vi "UHR-Fleezers Control (host) - 10.3.vi"() -> ()   [LabVIEW 2010] (continued)
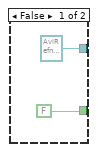
[diagram p2: hidden frame]
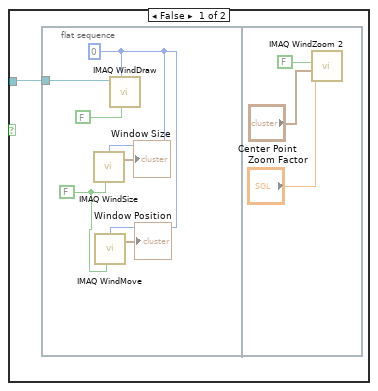
[diagram p5: hidden frame]
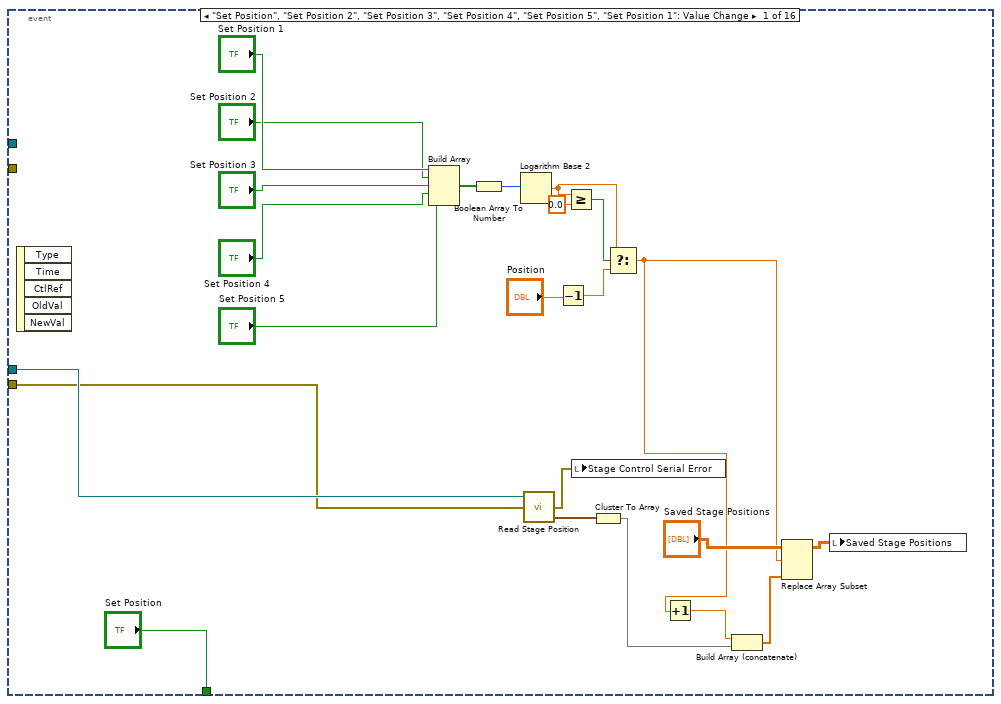
[diagram p11: hidden frame]
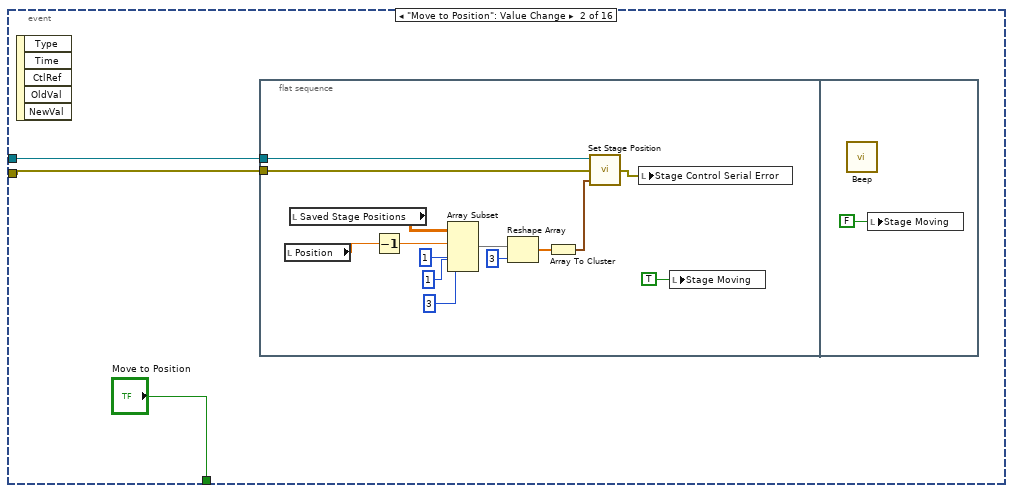
[diagram p12: hidden frame]
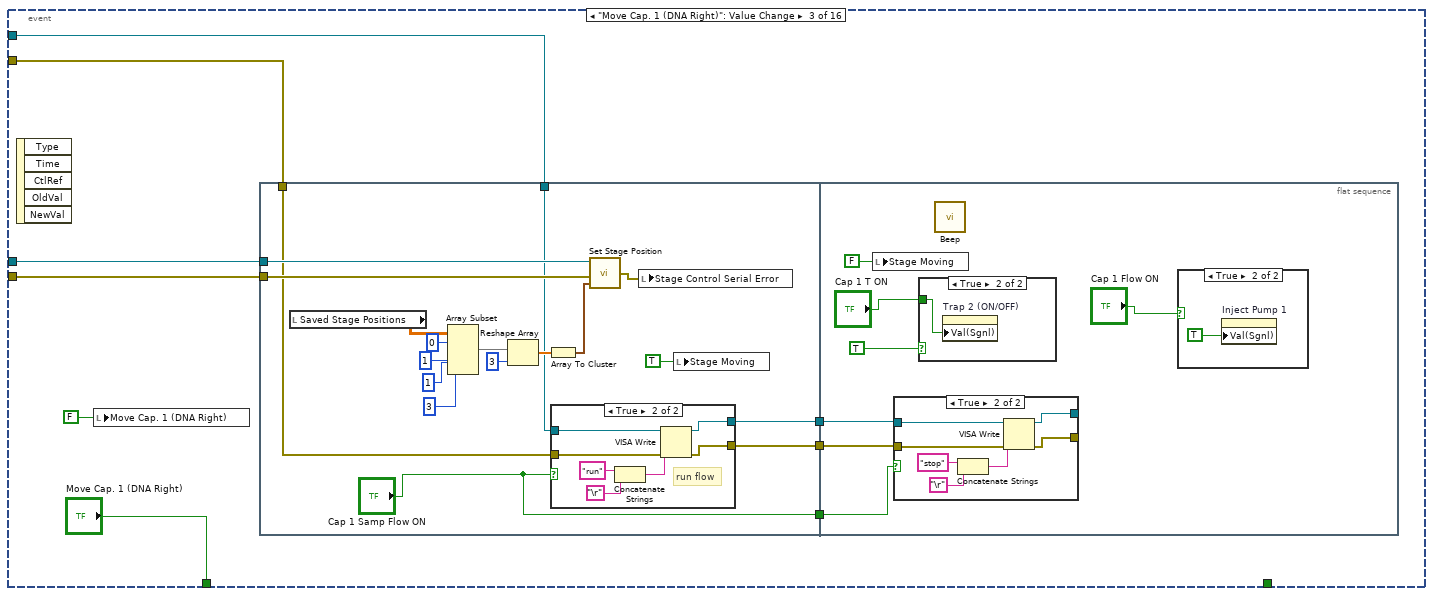
[diagram p13: hidden frame]
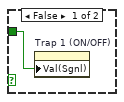
[diagram p17: hidden frame]
                          n1976 = local write "BD 2 Frequency 1 (MHz)"(w8359) -> ()
                          n1977 = local write "BD 1 Frequency 1 (MHz)"(w8361) -> ()
                        }
                      }
                    }
                    frame True {
                    }
                  }
                }
                event Mouse Up {
                  n1978 = event-data() -> ("Button"=w8364:u16)  [unwired: 8 out]
                  n1979 = case shown="3" w8364 {
                    tunnel: [FALSE TRUE] -> w8365
                    frame 0, Default {
                    }
                    frame 3 {
                      n1980 = local write "Manipulating Trap"(FALSE ("Manipulating Trap")) -> ()
                    }
                  }
                }
              }
            }
          }
        }
      }
      event Mouse Move {
        n1981 = event-data() -> ()  [unwired: 6 out]
      }
    }
    n1982 = local read "Stop All"() -> (w8186:bool)
    n1983 = node-c288() -> ()  [unwired: 2 out]
  }
  n1984 = disable-structure shown="Disabled" {
    frame Disabled {
      n1985 = flat-sequence "Video" {
        tunnel: [w8378] -> w8369
        tunnel: w8369 -> [w8419]
        frame #0 {
          n1986 = while {
            stop <- w8371 continue-if-true
            n1987 = call "Close Video Capture.vi"() -> ("error code OUT"=w8373:i32)
            n1988 = Equal?(x=w8373, y=0) -> (x = y?=w8371:bool)
          }
          n1989 = local write "Stop All"(FALSE ("Stop All")) -> ()
        }
        frame #1 {
          n1990 = call "DMR_Init.vi"() -> ()  [unwired: 3 out]
        }
        frame #2 {
          # "Setting the destination format to Mono8 makes sure that the image can be displayed in the intensity plot."
          n1991 = call "DMR_GetDevice.vi"("search string IN"="DE019116701") -> ("device handle OUT"=w8396:i32)  [unwired: 4 in, 2 out]
          n1992 = call "DMR_OpenDevice.vi"("device handle IN"=w8396) -> ("driver handle OUT"=w8379:i32)  [unwired: 4 out]
          n1993 = call "DMR_FindList.vi"("flags IN"=u32 0 ("flags"), "list name IN"="" ("String"), "list type IN"=T47."camera descriptions", "driver handle IN"=w8379) -> ("list handle OUT"=w8382:i32)  [unwired: 2 out]
          n1994 = call "DMR_FindList.vi"("flags IN"=u32 0 ("flags"), "list name IN"="Base", "list type IN"=T47."setting", "driver handle IN"=w8379) -> ("list handle OUT"=w8380:i32)  [unwired: 2 out]
          n1995 = call "OBJ_GetHandle.vi"("object name IN"="VideoStandard", "list handle IN"=w8382) -> ("object handle OUT"=w8376:i32)  [unwired: 3 out]
          n1996 = call "OBJ_GetHandle.vi"("object name IN"="PixelFormat", "list handle IN"=w8380) -> ("object handle OUT"=w8390:i32)  [unwired: 3 out]
          n1997 = call "OBJ_SetS.vi"("value index IN"=0, "value IN"="NTSC M", "object handle IN"=w8376) -> ()  [unwired: 2 out]
          n1998 = call "OBJ_SetS.vi"("value index IN"=0, "value IN"="Mono8" ("value"), "object handle IN"=w8390) -> ()  [unwired: 2 out]
          n1999 = call "OBJ_GetHandle.vi"("object name IN"="VideoChannel", "list handle IN"=w8380) -> ("object handle OUT"=w8386:i32)  [unwired: 3 out]
          n2000 = while {
            tunnel: [w8401] -> w8378
            tunnel: w8379 -> [w8398]
            stop <- w8399 continue-if-true
            n2001 = call "DMR_ImageRequestSingle.vi"("request control IN"=0, "driver handle IN"=w8398) -> ("error code OUT"=w8400:i32, "driver handle OUT"=w8401:i32)  [unwired: 2 out]
            n2002 = Equal To 0?(x=w8400) -> (x = 0?=w8399:bool)
          }
          n2003 = call "OBJ_SetI.vi"("value index IN"=0, "value IN"=3 ("Video channel"), "object handle IN"=w8386) -> ()  [unwired: 2 out]
        }
        frame #3 {
          w8407 = T17 0 items=["Grayscale (U8)", "Grayscale (I16)", "Grayscale (SGL)", "Complex (CSG)", "RGB (U32)", "HSL (U32)", "RGB (U64)"] ("Image Type")
          w8415 = T17 0 items=["Grayscale (U8)", "Grayscale (I16)", "Grayscale (SGL)", "Complex (CSG)", "RGB (U32)", "HSL (U32)", "RGB (U64)"] ("Image Type")
          n2004 = for "Create Greyscale map" {
            N: 256 -> [_]
            tunnel: [w8421] -> w8404 mode=indexing
            workers-P: _ -> [_]
            i -> [w8424]
            n2005 = To Unsigned Byte Integer(number=w8424) -> (unsigned 8bit integer=w8420:u8)
            n2006 = Join Numbers(hi=w8420, lo=w8420) -> ((hi.lo)=w8423:u16)
            n2007 = Join Numbers(hi=w8420, lo=w8420) -> ((hi.lo)=w8422:u16)
            n2008 = Join Numbers(hi=w8423, lo=w8422) -> ((hi.lo)=w8421:u32)
          }
          n2009 = call "IMAQ Create"("Image Name"="Scaled video", "Image Type"=w8407) -> ("New Image"=w8406:T2)  [unwired: 2 in, 2 out]
          n2010 = call "IMAQ Create"("Image Name"="Main video", "Image Type"=w8415) -> ("New Image"=w8416:T2)  [unwired: 2 in, 2 out]
          n2011 = node-c288(0 ("Processor")) -> (w8414:T23)  [unwired: 3 out]
          n2012 = Initialize Array(u32 0 ("Window Number (0...15)"), 480 ("dimension size"), 640 ("dimension size")) -> (w8409:u32[][])
          n2013 = timed-loop {
            tunnel: w8419 -> [w8441]
            tunnel: [w8440] -> w8418
            tunnel: w8416 -> [w8439]
            timing: w8414 -> [_]
            timing-out: [_] -> w8413
            tunnel: w8409 -> [w8428]
            tunnel: w8406 -> [w8426]
            tunnel: w8404 -> [w8425]
            stop <- w8427 stop-if-true
            # "This block performs the \nactual image capture."
            n2014 = node-c288() -> ()  [unwired: 2 out]
            n2015 = local read "Stop All"() -> (w8427:bool)
            n2016 = Reciprocal(x="Video Capture Rate (Hz)") -> (1/x=w8431:dbl)
            n2017 = Multiply(x=w8431, y=1000.0) -> (x*y=w8429:dbl)
            n2018 = call "DMR_ImageRequestWaitFor.vi"("queue number IN"=0, "timeout(ms) IN"=500, "driver handle IN"=w8441) -> ("error code OUT"=w8445:i32, "request number OUT"=w8442:i32, "driver handle OUT"=w8443:i32)
            n2019 = feedback #31(T48 refnum ("Avi Refnum")) -> (w8433:T48)
            n2020 = case shown="True" "New Video File" {
              tunnel: [T48 refnum ("Avi Refnum") w8462] -> w8435
              tunnel: [FALSE TRUE] -> w8436
              tunnel: w8433 -> [_ w8458]
              frame False {
              }
              frame True {
                n2021 = call "Create new save file.vi"("Ext"=".avi" ("string"), "Index In"="Video Index") -> ("Path Out"=w8454:path, "Index Out"=w8455:dbl)  [unwired: 1 in]
                "Path Out" <- w8454
                n2022 = Not Equal?(x=w8458, y=T48 refnum ("Avi Refnum")) -> (x != y?=w8459:bool)
                n2023 = Increment(x=w8455) -> (x+1=w8464:dbl)
                n2024 = case shown="True" w8459 {
                  tunnel: w8458 -> [_ w8465]
                  frame False {
                  }
                  frame True {
                    n2025 = call "IMAQ AVI Close"("Avi Refnum"=w8465) -> ()  [unwired: 1 in, 10 out]
                  }
                }
                n2026 = local write "Video Index"(w8464) -> ()
                n2027 = call "IMAQ AVI Create"("Frames Per Second"=u32 30, "AVI Path"=w8454) -> ("Avi Refnum"=w8462:T48)  [unwired: 5 in, 4 out]
              }
            }
            n2028 = Equal To 0?(x=w8445) -> (x = 0?=w8444:bool)
            n2029 = Select(t=w8435, s=w8436, f=w8433) -> (s? t:f=w8434:T48)
            n2030 = feedback-in #31(w8434) -> ()
            n2031 = case shown="True" w8444 {
              tunnel: w8443 -> [w8466 w8491]
              tunnel: w8442 -> [_ w8490]
              tunnel: [w8466 w8487] -> w8440
              tunnel: w8439 -> [_ w8471]
              tunnel: w8428 -> [_ w8475]
              tunnel: w8434 -> [_ w8473]
              tunnel: w8426 -> [_ w8468]
              tunnel: w8425 -> [_ w8467]
              frame False {
              }
              frame True {
                w8481 = u32 0 ("X-offset IN")
                n2032 = call "DMR_GetImageRequestBufferData.vi"("driver handle IN"=w8491, "request number IN"=w8490) -> ("width OUT"=w8480:i32, "height OUT"=w8479:i32, "driver handle OUT"=w8486:i32, "request number OUT"=w8485:i32, "bytes per pixel OUT"=w8482:i32)  [unwired: 13 out]
                n2033 = call "DMR_GetImageRequestBufferImageData.vi"("driver handle IN"=w8486, "request number IN"=w8485, "bytes per pixel IN"=w8482, "X-offset IN"=w8481, "Y-offset IN"=w8481, "height IN"=w8479, "width IN"=w8480) -> ("driver handle OUT"=w8484:u32, "request number OUT"=w8483:u32, "image OUT"=w8476:u32[][])  [unwired: 10 out]
                n2034 = call "DMR_ImageRequestUnlock.vi"("request number IN"=w8483, "driver handle IN"=w8484) -> ("driver handle OUT"=w8489:i32)  [unwired: 1 in, 2 out]
                n2035 = case shown="True" "Averaging" {
                  tunnel: w8476 -> [w8527 w8532]
                  tunnel: [w8527 w8531] -> w8472
                  tunnel: w8475 -> [_ w8529]
                  frame False {
                  }
                  frame True {
                    (unwired) 1
                    w8537 = 1
                    n2036 = feedback #32(w8529) -> (w8528:u32[][])
                    n2037 = Add(x=w8532, y=w8528) -> (x+y=w8533:u32[][])
                    n2038 = Select(t=w8529, s="Reset Averaging", f=w8533) -> (s? t:f=w8535:u32[][])
                    n2039 = feedback-in #32(w8535) -> ()
                    n2040 = feedback #33(w8537) -> (w8530:i32)
                    n2041 = Divide(x=w8533, y=w8530) -> (x/y=w8534:dbl[][])
                    n2042 = Increment(x=w8530) -> (x+1=w8538:i32)
                    n2043 = To Unsigned Long Integer(number=w8534) -> (unsigned 32bit integer=w8531:u32[][])
                    n2044 = Select(t=w8537, s="Reset Averaging", f=w8538) -> (s? t:f=w8536:i32)
                    n2045 = feedback-in #33(w8536) -> ()
                  }
                }
                n2046 = call "DMR_ImageRequestSingle.vi"("request control IN"=0, "driver handle IN"=w8489) -> ("driver handle OUT"=w8487:i32)  [unwired: 3 out]
                n2047 = disable-structure shown="Disabled" {
                  disable-tunnel: w8472 -> [w8504 _]
                  disable-tunnel: w8468 -> [w8503 _]
                  frame Disabled {
                    n2048 = To Double Precision Float(number=w8504) -> (double precision float=w8502:dbl[][])
                    n2049 = In Range and Coerce(upper limit="Intensity Upper", x=w8502, lower limit="Intensity Lower") -> (coerced(x)=w8501:dbl[][])  [unwired: 1 out]
                    n2050 = Subtract(x="Intensity Upper", y="Intensity Lower") -> (x-y=w8498:dbl)
                    n2051 = Subtract(x=w8501, y="Intensity Lower") -> (x-y=w8499:dbl[][])
                    n2052 = Divide(x=w8499, y=w8498) -> (x/y=w8500:dbl[][])
                    n2053 = Multiply(x=255.0, y=w8500) -> (x*y=w8496:dbl[][])
                    n2054 = To Unsigned Byte Integer(number=w8496) -> (unsigned 8bit integer=w8505:u8[][])
                    n2055 = call "IMAQ ArrayToImage"("Image Pixels (U8)"=w8505, "Image"=w8503) -> ("Image Out"=w8492:T2)  [unwired: 4 in, 5 out]
                    n2056 = First Call?() -> (First Call?: T/F=w8493:bool)
                    n2057 = case shown="True" w8493 {
                      tunnel: w8492 -> [w8506 w8517]
                      frame False {
                        n2058 = flat-sequence {
                          tunnel: w8506 -> [w8512]
                          frame #0 {
                            w8509 = FALSE ("Get/Set Status? (Set)")
                            w8508 = 0 ("Window Number (0...15)")
                            n2059 = call "IMAQ WindSize"("Get/Set Status? (Set)"=w8509, "Window Number"=w8508) -> ("Width & Height out"=→"Window Size":cluster{"Width":i32, "Height":i32})  [unwired: 4 in, 2 out]
                            n2060 = call "IMAQ WindMove"("Window Number (0...15)"=w8508, "Get/Set Status? (Set)"=w8509) -> ("Coordinates (screen)"=→"Window Position":cluster{"X Position":i32, "Y Position":i32})  [unwired: 3 in, 1 out]
                            n2061 = call "IMAQ WindDraw"("Resize to Image Size? (Y)"=FALSE, "Window Number (0...15)"=w8508, "Image"=w8512) -> ()  [unwired: 7 in, 2 out]
                          }
                          frame #1 {
                            n2062 = call "IMAQ WindZoom 2"("Center Point"="Center Point", "Zoom to Fit? (False)"=FALSE, "Zoom Factor"="Zoom Factor") -> ()  [unwired: 5 in, 4 out]
                          }
                        }
                      }
                      frame True {
                        n2063 = flat-sequence {
                          tunnel: w8517 -> [w8520]
                          tunnel: [w8518] -> w8516
                          tunnel: w8516 -> [w8522]
                          frame #0 {
                            w8519 = TRUE ("Resize to Image Size? (Y)")
                            w8518 = 0 ("Window Number (0...15)")
                            n2064 = call "IMAQ WindNonTearing"("Window Number"=w8518, "NonTearing? (True)"=w8519) -> ()  [unwired: 8 in, 2 out]
                            n2065 = call "IMAQ WindDraw"("Resize to Image Size? (Y)"=w8519, "Window Number (0...15)"=w8518, "Image"=w8520) -> ()  [unwired: 7 in, 2 out]
                          }
                          frame #1 {
                            n2066 = call "IMAQ WindSize"("Scrollbars? (N)"=FALSE, "Width & Height"="Initial Window Size", "Window Number"=w8522) -> ()  [unwired: 3 in, 3 out]
                            n2067 = call "IMAQ WindMove"("Window Number (0...15)"=w8522, "Coordinates (screen)"="Initial Window Position") -> ()  [unwired: 3 in, 2 out]
                          }
                        }
                      }
                    }
                  }
                  frame Enabled {
                  }
                }
                n2068 = To Unsigned Byte Integer(number=w8472) -> (unsigned 8bit integer=w8470:u8[][])
                n2069 = call "IMAQ ArrayToImage"("Image Pixels (U8)"=w8470, "Image"=w8471) -> ("Image Out"=w8469:T2)  [unwired: 4 in, 5 out]
                "Primary Video Display" <- w8469
                n2070 = case shown="True" "Save Video" {
                  tunnel: w8473 -> [_ w8526]
                  tunnel: w8469 -> [_ w8525]
                  frame False {
                  }
                  frame True {
                    n2071 = call "IMAQ AVI Write Frame"("Image"=w8525, "Avi Refnum"=w8526) -> ()  [unwired: 2 in, 8 out]
                  }
                }
                n2072 = case shown="True" "Save Image" {
                  tunnel: w8470 -> [_ w8541]
                  tunnel: w8467 -> [_ w8540]
                  frame False {
                  }
                  frame True {
                    n2073 = call <vilib>:"Flatten Pixmap.vi"("colors"=w8540, "8-bit pixmap"=w8541) -> ("image data"=w8547:T49)  [unwired: 4 in, 5 out]
                    n2074 = call "Create new save file.vi"("Insert"="video_frame_" ("string"), "Ext"=".bmp" ("string"), "Index In"="Image Index") -> ("Path Out"=w8543:path, "Index Out"=w8548:dbl)
                    n2075 = Increment(x=w8548) -> (x+1=w8542:dbl)
                    n2076 = local write "Image Index"(w8542) -> ()
                    n2077 = call <vilib>:"Write BMP File.vi"("image data"=w8547, "path to BMP file"=w8543) -> ()  [unwired: 1 in, 9 out]
                  }
                }
              }
            }
            n2078 = node-c288(w8429) -> ()  [unwired: 1 out]
          }
          n2079 = node-c288(w8413) -> ()  [unwired: 1 out]
          n2080 = call "DMR_CloseDevice.vi"("driver handle IN"=w8418) -> ()  [unwired: 1 in, 4 out]
        }
        frame #4 {
          n2081 = call "DMR_Close.vi"() -> ()  [unwired: 1 out]
        }
      }
    }
    frame Enabled {
    }
  }
  n2082 = timed-loop "Oscillate AOD (debugging)" {
    tunnel: w8 -> [w8554]
    tunnel: [w8553] -> w52
    timing: w47 -> [_]
    timing-out: [_] -> w46
    stop <- w8553 stop-if-true
    n2083 = node-c288() -> ()  [unwired: 2 out]
    n2084 = event shown="[0] \"Oscillate Set 1\", \"Fish for Tether\": Value Change" {
      selector: _ -> [_ _ _]
      dyn-events: _ -> [_ _ _]
      timeout: _ -> [_ _ _]
      tunnel: w8554 -> [w8561 _ _]
      tunnel: [FALSE ("Stop All") _ w8830] -> w8553
      event "Oscillate Set 1", "Fish for Tether": Value Change {
        n2085 = event-data() -> ()  [unwired: 6 out]
        n2086 = local read "Oscillate Set 1"() -> (w8560:bool)
        n2087 = Or(x=w8560, y="Fish for Tether") -> (x .or. y?=w8558:bool)
        n2088 = case shown="True" w8558 {
          tunnel: w8561 -> [_ w8564]
          tunnel: "Fish for Tether" -> [_ w8563]
          frame False {
          }
          frame True {
            n2089 = case shown="False" w8563 {
              frame False {
              }
              frame True {
                n2090 = local write "Scan axis 2"(TRUE) -> ()
                n2091 = local write "Tether"(FALSE ("Tether")) -> ()
              }
            }
            n2092 = node-c288(i64 50 ("Period")) -> (w8566:T23)  [unwired: 3 out]
            n2093 = timed-loop "Oscillate AOD" {
              timing: w8566 -> [_]
              timing-out: [_] -> w8565
              tunnel: w8564 -> [w8576]
              tunnel: w8563 -> [w8575]
              i -> [w8578]
              stop <- w8574 stop-if-true
              n2094 = node-c288() -> (w8577:i64)  [unwired: 1 out]
              n2095 = flat-sequence {
                tunnel: w8578 -> [w8605]
                tunnel: w8577 -> [w8604]
                tunnel: w8576 -> [w8585]
                tunnel: w8575 -> [w8588]
                tunnel: [w8588] -> w8573
                tunnel: [w8587] -> w8572
                tunnel: [w8584] -> w8571
                tunnel: [w8581] -> w8569
                tunnel: w8573 -> [w8641]
                tunnel: w8572 -> [w8639]
                tunnel: w8571 -> [w8638]
                tunnel: [w8637] -> w8570
                tunnel: w8569 -> [w8636]
                tunnel: [w8705] -> w8574
                tunnel: w8570 -> [w8703]
                frame #0 {
                  n2096 = Divide(x=w8604, y=i64 1000) -> (x/y=w8599:dbl)
                  n2097 = Multiply(x=w8599, y=w8605) -> (x*y=w8601:dbl)
                  n2098 = Multiply(x="Osc. freq. (Hz)", y=6.283185307179586) -> (x*y=w8602:dbl)
                  n2099 = Multiply(x=w8602, y=w8601) -> (x*y=w8583:dbl)
                  n2100 = local read "BD 1 Frequency 2 (MHz)"() -> (w8586:dbl)
                  n2101 = local read "BD 1 Frequency 1 (MHz)"() -> (w8579:dbl)
                  n2102 = case shown="False" w8588 {
                    tunnel: w8583 -> [w8611 w8617]
                    tunnel: w8586 -> [_ w8628]
                    tunnel: [w8608 w8623] -> w8589
                    tunnel: [FALSE w8620] -> w8584
                    tunnel: [0.0 w8613] -> w8581
                    tunnel: w8579 -> [_ w8612]
                    frame False {
                      n2103 = Sine(x=w8611) -> (sin(x)=w8609:dbl)
                      n2104 = Multiply(x=w8609, y="Osc. amp. (MHz)") -> (x*y=w8608:dbl)
                    }
                    frame True {
                      n2105 = Cosine(x=w8617) -> (cos(x)=w8631:dbl)
                      n2106 = Subtract(x=w8628, y=w8612) -> (x-y=w8627:dbl)
                      n2107 = Decrement(x=w8631) -> (x-1=w8630:dbl)
                      n2108 = Subtract(x=w8627, y="Closest Delta (MHz)") -> (x-y=w8624:dbl)
                      n2109 = Divide(x=w8630, y=-2.0) -> (x/y=w8625:dbl)
                      n2110 = Multiply(x=w8625, y=w8624) -> (x*y=w8623:dbl)
                      n2111 = local read "Vec Mean of T1 T2"() -> (w8619:dbl[])
                      n2112 = Greater?(x=w8619, y="Stop F (pN)") -> (0:w8621:bool[])
                      n2113 = Or Array Elements(Boolean array=w8621) -> (logical OR=w8620:bool)
                      n2114 = Divide(x=w8617, y=6.283185307179586) -> (x/y=w8616:dbl)
                      n2115 = Round Toward +Infinity(x=w8616) -> (ceil(x): smallest int >= x=w8613:dbl)
                      "Attempts" <- w8613
                      n2116 = Greater?(x=w8613, y="Attempt Limit") -> (0:w8615:bool)
                      n2117 = case shown="True" w8615 {
                        frame False {
                        }
                        frame True {
                          n2118 = local write "Fish for Tether"(FALSE ("Fish for Tether")) -> ()
                          n2119 = call <vilib>:"Beep.vi"() -> ()  [unwired: 3 in, 9 out]
                          n2120 = local read "Messages"() -> (w8633:string)
                          n2121 = call "Update messages.vi"("Message to add"="Tether fishing timeout." ("Messages"), "Old message string"=w8633) -> ("New message string"=→"Messages":string)
                        }
                      }
                    }
                  }
                  n2122 = local read "BD 2 Frequency 1 (MHz)"() -> (w8590:dbl)
                  n2123 = Select(t=w8579, s="Scan axis 2", f=w8590) -> (s? t:f=w8593:dbl)
                  n2124 = Add(x=w8589, y=w8593) -> (x+y=w8587:dbl)
                  n2125 = Select(t=w8587, s="Scan axis 2", f=w8579) -> (s? t:f=w8580:dbl)
                  n2126 = Select(t=w8590, s="Scan axis 2", f=w8587) -> (s? t:f=w8595:dbl)
                  n2127 = local read "Y RF Frequency Limits (MHz)"() -> (w8591:T16)
                  n2128 = local read "X RF Frequency Limits (MHz)"() -> (w8592:T16)
                  n2129 = local read "BD 1 Frequency 3 (MHz)"() -> (w8598:dbl)
                  n2130 = local read "BD 2 Frequency 2 (MHz)"() -> (w8597:dbl)
                  n2131 = local read "BD 2 Frequency 3 (MHz)"() -> (w8596:dbl)
                  n2132 = call "set RF board frequency - interlace.vi"("Board 2 Frequency Limits"=w8591, "Board 1 Frequency Limits"=w8592, "FPGA VI Reference In"=w8585, "Board 2 Frequency 3 (MHz)"=w8596, "Board 1 Frequency 3 (MHz)"=w8598, "Board 2 Frequency 2 (MHz)"=w8597, "Board 2 Frequency 1 (MHz)"=w8595, "Board 1 Frequency 2 (MHz)"=w8586, "Board 1 Frequency 1  (MHz)"=w8580) -> ()  [unwired: 1 in, 2 out]
                }
                frame #1 {
                  n2133 = And(x=w8641, y=w8638) -> (x .and. y?=w8640:bool)
                  n2134 = case "Only if were fishing and now formed tether" shown="False" w8640 {
                    tunnel: w8639 -> [w8643 w8655]
                    tunnel: [w8642 w8654] -> w8637
                    tunnel: w8636 -> [_ w8650]
                    frame False {
                      n2135 = local read "Fish for Tether"() -> (w8642:bool)
                      n2136 = case shown="False" w8642 {
                        tunnel: w8643 -> [_ _]
                        frame False {
                        }
                        frame True {
                        }
                      }
                    }
                    frame True {
                      w8654 = FALSE ("Fish for Tether")
                      n2137 = call <vilib>:"Beep.vi"() -> ()  [unwired: 3 in, 9 out]
                      n2138 = Number To Decimal String(number=w8650, width (-)=i16 1) -> (decimal integer string=w8648:string)
                      n2139 = case shown="\"1\", Default" "Then..." {
                        selector: "Then..." -> [_ w8658]
                        tunnel: w8655 -> [w8657 _]
                        frame "1", Default {
                          n2140 = property on="BD 1 Frequency 1 (MHz)" class="DigNum (strict)"("Val(Sgnl)"=w8657) -> ()  [unwired: 2 in, 2 out]
                        }
                        frame "2", "3", "4", "5", "6" {
                          n2141 = flat-sequence {
                            tunnel: w8658 -> [w8660]
                            frame #0 {
                              n2142 = property on="Trap Delta (MHz)" class="DigNum (strict)"("Val(Sgnl)"="Move to Delta 1 (MHz)") -> ()  [unwired: 2 in, 2 out]
                            }
                            frame #1 {
                              n2143 = case shown="\"5\", \"6\"" w8660 {
                                selector: w8660 -> [w8663 w8673 _]
                                frame "3", "4" {
                                n2144 = flat-sequence {
                                tunnel: w8663 -> [w8664]
                                tunnel: [w8664] -> w8661
                                tunnel: [w8666] -> w8662
                                tunnel: w8661 -> [w8666]
                                tunnel: w8662 -> [w8670]
                                frame #0 {
                                n2145 = property on="Green Laser ON/Interlacing" class="Bool (strict)"("Val(Sgnl)"=TRUE ("Value (Signaling)")) -> ()  [unwired: 2 in, 2 out]
                                }
                                frame #1 {
                                n2146 = Multiply(x="Wait Before Save (s)", y=u32 1000 ("x")) -> (x*y=w8668:u32)
                                n2147 = Wait (ms)(milliseconds to wait=w8668) -> ()  [unwired: 1 out]
                                }
                                frame #2 {
                                n2148 = property on="Start Saving" class="Bool (strict)"("Value"=TRUE ("Start Saving")) -> ()  [unwired: 2 in, 2 out]
                                n2149 = case shown="\"4\"" w8670 {
                                frame Default {
                                }
                                frame "4" {
                                n2150 = property on="Fl. Triggered..." class="Bool (strict)"("Val(Sgnl)"=TRUE ("Value (Signaling)")) -> ()  [unwired: 2 in, 2 out]
                                }
                                }
                                }
                                }
                                }
                                frame "5", "6" {
                                n2151 = stacked-sequence {
                                tunnel: w8673 -> [_ _ _ _ _ _ _ _ w8690 _ _]
                                frame #0 {
                                n2152 = Replace Array Subset(array=u32[] [0] ("Index Values"), new element="Raster Set Upon Tether", index=0) -> (w8674:u32[])
                                n2153 = property on="Saved AOD Raster Scan Parameter Sets" class="Arr (strict)"("Index Values"=w8674) -> ()  [unwired: 2 in, 2 out]
                                }
                                frame #1 {
                                n2154 = Wait (ms)(milliseconds to wait=u32 500) -> ()  [unwired: 1 out]
                                }
                                frame #2 {
                                n2155 = property on="Load parameters" class="Bool (strict)"("Val(Sgnl)"=TRUE ("Value (Signaling)")) -> ()  [unwired: 2 in, 2 out]
                                }
                                frame #3 {
                                n2156 = Wait (ms)(milliseconds to wait=u32 500) -> ()  [unwired: 1 out]
                                }
                                frame #4 {
                                n2157 = property on="Trap Raster Scan" class="Bool (strict)"("Val(Sgnl)"=TRUE ("Value (Signaling)")) -> ()  [unwired: 2 in, 2 out]
                                }
                                frame #5 {
                                n2158 = Wait (ms)(milliseconds to wait=u32 2000) -> ()  [unwired: 1 out]
                                }
                                frame #6 {
                                n2159 = while {
                                stop <- w8685 stop-if-true
                                n2160 = local read "Raster Scanning..."() -> (w8684:bool)
                                n2161 = local read "Saving..."() -> (w8687:bool)
                                n2162 = Wait (ms)(milliseconds to wait=u32 100) -> ()  [unwired: 1 out]
                                n2163 = Not(x=w8687) -> (.not. x?=w8686:bool)
                                n2164 = Not(x=w8684) -> (.not. x?=w8683:bool)
                                n2165 = And(x=w8686, y=w8683) -> (x .and. y?=w8685:bool)
                                }
                                }
                                frame #7 {
                                n2166 = property on="Trap Delta (MHz)" class="DigNum (strict)"("Val(Sgnl)"="Move to Delta 2 (MHz)") -> ()  [unwired: 2 in, 2 out]
                                }
                                frame #8 {
                                n2167 = local read "Tether"() -> (w8691:bool)
                                n2168 = case shown="True" w8691 {
                                tunnel: w8690 -> [_ w8692]
                                frame False {
                                }
                                frame True {
                                n2169 = flat-sequence {
                                tunnel: w8692 -> [w8694]
                                frame #0 {
                                n2170 = Wait (ms)(milliseconds to wait=u32 500) -> ()  [unwired: 1 out]
                                }
                                frame #1 {
                                n2171 = case shown="\"6\"" w8694 {
                                frame Default {
                                }
                                frame "6" {
                                n2172 = property on="Green Laser ON/Interlacing" class="Bool (strict)"("Val(Sgnl)"=TRUE ("Green Laser ON/Interlacing")) -> ()  [unwired: 2 in, 2 out]
                                }
                                }
                                }
                                frame #2 {
                                n2173 = Wait (ms)(milliseconds to wait=u32 500) -> ()  [unwired: 1 out]
                                }
                                frame #3 {
                                n2174 = local write "Start Saving"("Save at end (5, 6)") -> ()
                                }
                                }
                                }
                                }
                                }
                                frame #9 {
                                n2175 = local read "Bead Sep. Int. Time (s)"() -> (w8700:dbl)
                                n2176 = Multiply(x=w8700, y=1000.0) -> (x*y=w8699:dbl)
                                n2177 = Wait (ms)(milliseconds to wait=w8699) -> ()  [unwired: 1 out]
                                }
                                frame #10 {
                                n2178 = property on="Rescale on Mean" class="Bool (strict)"("Val(Sgnl)"=TRUE ("Value (Signaling)")) -> ()  [unwired: 2 in, 2 out]
                                }
                                }
                                }
                                frame "2", Default {
                                }
                              }
                            }
                          }
                        }
                      }
                      n2179 = Concatenate Strings("Formed tether in ", w8648, " attempt(s)." ("string")) -> (w8645:string)
                      n2180 = local read "Messages"() -> (w8652:string)
                      n2181 = local write "Fish for Tether"(w8654) -> ()
                      n2182 = call "Update messages.vi"("Message to add"=w8645, "Old message string"=w8652) -> ("New message string"=w8651:string)
                      n2183 = local write "Messages"(w8651) -> ()
                      n2184 = Get Date/Time In Seconds() -> (seconds since 1Jan1904=→"Time tether formed":timestamp)
                      "Tether" <- "Tether Alarm?"
                    }
                  }
                }
                frame #2 {
                  n2185 = local read "Oscillate Set 1"() -> (w8704:bool)
                  n2186 = local read "Stop All"() -> (w8706:bool)
                  n2187 = Not Or(1:w8703, 2:w8704) -> (0:w8702:bool)
                  n2188 = Compound Arithmetic op=OR(w8706, w8702) -> (w8705:bool)
                }
              }
              n2189 = node-c288() -> ()  [unwired: 2 out]
            }
            n2190 = node-c288(w8565) -> ()  [unwired: 1 out]
          }
        }
      }
      event "Fl. Triggered...": Value Change {
        n2191 = event-data() -> ()  [unwired: 7 out]
        n2192 = case shown="True" "Fl. Triggered..." {
          frame False {
          }
          frame True {
            n2193 = node-c288() -> (w8718:T23)  [unwired: 4 out]
            n2194 = timed-loop {
              timing: w8718 -> [_]
              timing-out: [_] -> w8717
              tunnel: "Action" -> [w8722]
              shift-right: [w8719] -> _
              shift-left: u8 255 -> [w8721]
              stop <- w8723 stop-if-true
              n2195 = node-c288() -> ()  [unwired: 2 out]
              n2196 = flat-sequence {
                tunnel: w8722 -> [w8735]
                tunnel: w8721 -> [w8732]
                tunnel: [w8731] -> w8720
                tunnel: [w8821] -> w8723
                tunnel: w8720 -> [w8820]
                tunnel: [w8820] -> w8719
                frame #0 {
                  n2197 = local read "Delta Fl. 2"() -> (w8726:dbl)
                  n2198 = local read "Delta Fl. 1"() -> (w8727:dbl)
                  n2199 = Select(t=w8727, s="APD to Watch", f=w8726) -> (s? t:f=w8725:dbl)
                  n2200 = Multiply(x="Fl. Delta Thresh. (kHz)", y=1000.0) -> (x*y=w8734:dbl)
                  n2201 = Greater?(x=w8725, y=w8734) -> (0:w8729:bool)
                  n2202 = Or(x="Force Yank", y=w8729) -> (x .or. y?=w8730:bool)
                  n2203 = case shown="True" w8730 {
                    tunnel: w8735 -> [_ w8745]
                    tunnel: w8732 -> [w8737 w8741]
                    tunnel: [w8737 w8738] -> w8731
                    frame False {
                    }
                    frame True {
                      n2204 = flat-sequence {
                        tunnel: w8742 -> [w8751]
                        tunnel: [w8751] -> w8746
                        tunnel: w8745 -> [w8750]
                        tunnel: [w8750] -> w8744
                        tunnel: [w8749] -> w8743
                        tunnel: w8741 -> [w8748]
                        tunnel: [w8747] -> w8740
                        tunnel: w8746 -> [w8776]
                        tunnel: w8744 -> [w8775]
                        tunnel: w8743 -> [w8774]
                        tunnel: w8740 -> [w8773]
                        tunnel: [w8773] -> w8739
                        tunnel: w8739 -> [w8818]
                        tunnel: [w8818] -> w8738
                        frame #0 {
                          n2205 = call <vilib>:"Beep.vi"() -> ()  [unwired: 3 in, 9 out]
                          n2206 = local write "Waiting"(FALSE ("Waiting")) -> ()
                          n2207 = Increment(x=w8748) -> (x+1=w8747:u8)
                          n2208 = case shown="\"Yank\"" w8750 {
                            tunnel: w8747 -> [_ _ w8757]
                            frame "Image" {
                              n2209 = property on="Confocal Image" class="Bool (strict)"("Val(Sgnl)"=TRUE ("Value (Signaling)")) -> ()  [unwired: 2 in, 2 out]
                            }
                            frame "Alarm", Default {
                            }
                            frame "Yank" {
                              n2210 = flat-sequence {
                                tunnel: w8757 -> [w8760]
                                tunnel: [w8759] -> w8756
                                tunnel: ["N Array El"] -> w8755
                                tunnel: w8756 -> [w8770]
                                tunnel: w8755 -> [w8766]
                                frame #0 {
                                n2211 = Multiply(x="Yank Delay (s)", y=1000.0) -> (x*y=w8763:dbl)
                                n2212 = Quotient & Remainder(x=w8760, y="N Array El") -> (x-y*floor(x/y)=w8759:u8)  [unwired: 1 out]
                                n2213 = Wait (ms)(milliseconds to wait=w8763) -> ()  [unwired: 1 out]
                                }
                                frame #1 {
                                n2214 = Random Number (0-1)() -> (number: 0 to 1=w8767:dbl)
                                n2215 = Multiply(x=w8766, y=w8767) -> (x*y=w8765:dbl)
                                n2216 = Round Toward -Infinity(1:w8765) -> (0:w8764:dbl)
                                n2217 = Select(t=w8764, s="Random Choice", f=w8770) -> (s? t:f=w8768:dbl)
                                n2218 = Index Array(array="Yank to Delta Array (MHz)", index=w8768) -> (element=w8771:dbl)
                                n2219 = property on="Trap Delta (MHz)" class="DigNum (strict)"("Val(Sgnl)"=w8771) -> ()  [unwired: 2 in, 2 out]
                                }
                              }
                            }
                          }
                          n2220 = local read "Time (s)"() -> (w8749:dbl)
                          "Fl. High" <- TRUE ("Yanking")
                        }
                        frame #1 {
                          n2221 = node-c288() -> (w8778:T23)  [unwired: 4 out]
                          n2222 = timed-loop {
                            timing: w8778 -> [_]
                            timing-out: [_] -> w8777
                            tunnel: w8776 -> [w8794]
                            tunnel: w8775 -> [w8792]
                            tunnel: w8774 -> [w8791]
                            stop <- w8793 stop-if-true
                            n2223 = node-c288() -> ()  [unwired: 2 out]
                            n2224 = local read "Fl. Delta Thresh. (kHz)"() -> (w8786:dbl)
                            n2225 = local read "Fl. Triggered..."() -> (w8795:bool)
                            n2226 = local read "Delta Fl. 1"() -> (w8782:dbl)
                            n2227 = local read "Delta Fl. 2"() -> (w8780:dbl)
                            n2228 = local read "Stop All"() -> (w8789:bool)
                            n2229 = local read "APD to Watch"() -> (w8781:bool)
                            n2230 = Select(t=w8782, s=w8781, f=w8780) -> (s? t:f=w8779:dbl)
                            n2231 = Not(x=w8795) -> (.not. x?=w8790:bool)
                            n2232 = Multiply(x=w8786, y=1000.0) -> (x*y=w8785:dbl)
                            n2233 = Negate(x=w8785) -> (-x=w8784:dbl)
                            n2234 = Less?(x=w8779, y=w8784) -> (x < y?=w8788:bool)
                            n2235 = Compound Arithmetic op=OR(w8788, w8789, w8790, "Force Reset") -> (w8793:bool)
                            n2236 = case shown="True" w8793 {
                              tunnel: w8794 -> [_ w8806]
                              tunnel: w8792 -> [_ w8805]
                              tunnel: w8791 -> [_ w8803]
                              frame False {
                              }
                              frame True {
                                n2237 = case shown="\"Yank\"" w8805 {
                                tunnel: w8806 -> [_ w8807]
                                frame "Image", Default {
                                }
                                frame "Yank" {
                                n2238 = flat-sequence {
                                tunnel: [w8812] -> w8808
                                tunnel: w8807 -> [w8812]
                                tunnel: w8808 -> [w8813]
                                frame #0 {
                                n2239 = local read "Yank Delay (s)"() -> (w8811:dbl)
                                n2240 = Multiply(x=w8811, y=1000.0) -> (x*y=w8809:dbl)
                                n2241 = Wait (ms)(milliseconds to wait=w8809) -> ()  [unwired: 1 out]
                                }
                                frame #1 {
                                n2242 = property on="Trap Delta (MHz)" class="DigNum (strict)"("Val(Sgnl)"=w8813) -> ()  [unwired: 2 in, 2 out]
                                }
                                }
                                }
                                }
                                n2243 = local read "Time (s)"() -> (w8804:dbl)
                                n2244 = Subtract(x=w8804, y=w8803) -> (x-y=w8800:dbl)
                                "Duration (s)" <- w8800
                                n2245 = Number To Decimal String(number=w8800, width (-)=i16 0) -> (decimal integer string=w8798:string)
                                n2246 = Concatenate Strings(w8798, " s fluorescence event." ("string")) -> (w8796:string)
                                n2247 = local read "Messages"() -> (w8802:string)
                                n2248 = call "Update messages.vi"("Message to add"=w8796, "Old message string"=w8802) -> ("New message string"=w8801:string)
                                n2249 = call <vilib>:"Beep.vi"() -> ()  [unwired: 3 in, 9 out]
                                n2250 = local write "Messages"(w8801) -> ()
                              }
                            }
                            n2251 = node-c288() -> ()  [unwired: 2 out]
                          }
                          n2252 = node-c288(w8777) -> ()  [unwired: 1 out]
                        }
                        frame #2 {
                          n2253 = local write "Fl. High"(FALSE ("Yanking")) -> ()
                        }
                      }
                      n2254 = local read "Trap Delta (MHz)"() -> (w8742:dbl)
                    }
                  }
                }
                frame #1 {
                  n2255 = local read "Stop All"() -> (w8824:bool)
                  n2256 = local read "Fl. Triggered..."() -> (w8822:bool)
                  n2257 = Not(x=w8822) -> (.not. x?=w8823:bool)
                  n2258 = Or(x=w8823, y=w8824) -> (x .or. y?=w8821:bool)
                  n2259 = Not(x=w8821) -> (.not. x?=→"Waiting":bool)
                }
              }
              n2260 = node-c288() -> ()  [unwired: 2 out]
            }
            n2261 = node-c288(w8717) -> ()  [unwired: 1 out]
          }
        }
      }
      event "Stop All": Value Change {
        n2262 = event-data() -> ()  [unwired: 7 out]
        n2263 = local read "Stop All"() -> (w8830:bool)
      }
    }
    n2264 = node-c288() -> ()  [unwired: 2 out]
  }
  n2265 = node-c288(w48) -> ()  [unwired: 1 out]
  n2266 = node-c288(w36) -> ()  [unwired: 1 out]
  n2267 = VISA Close(VISA resource name=w39, error in (no error)=w38) -> (error out=w92:errorcluster)
  n2268 = node-c288(w50) -> ()  [unwired: 1 out]
  n2269 = call <vilib>:"Simple Error Handler.vi"("error in (no error)"=w92) -> ()  [unwired: 1 in, 8 out]
  n2270 = node-c288(w46) -> ()  [unwired: 1 out]
  n2271 = node-c288(w147) -> ()  [unwired: 1 out]
  n2272 = flat-sequence {
    tunnel: w242 -> [w8834]
    tunnel: w244 -> [w8835]
    tunnel: [w8833] -> w223
    tunnel: [w8832] -> w222
    tunnel: w204 -> [_]
    tunnel: w202 -> [_]
    tunnel: w155 -> [_]
    tunnel: w52 -> [_]
    tunnel: w223 -> [w8895]
    tunnel: w222 -> [w8896]
    frame #0 {
      w8831 = FALSE ("AI to FIFO")
      n2273 = xnode "Read/Write Control"("FPGA VI Reference In"=w8835, "error in"=w8834, "AI to FIFO"=w8831, "APD to FIFO"=w8831) -> ("FPGA VI Reference Out"=w8833:T19, "error out"=w8832:errorcluster)
    }
    frame #1 {
      n2274 = xnode "Close FPGA VI Reference"("FPGA VI Reference In"=w8895, "error in"=w8896) -> ("error out"=→"error out":errorcluster)
    }
  }
